vi "HFRR ADV v044.vi"() -> ()   [LabVIEW 2025] (continued)
                  selector: w401 -> [_ w412]
                  frame False {
                    w408 = TRUE ("PAUSE")
                    n303 = call "ELAPSED TIMER VI - abort test.vi"("RESET"=w408, "PAUSE"=w408) -> ()  [unwired: 7 in, 3 out]
                  }
                  frame True {
                    n304 = Not(x=w412) -> (.not. x?=w411:bool)
                    n305 = call "ELAPSED TIMER VI - abort test.vi"("TARGET"=60.0, "RESET"=w411, "PAUSE"=FALSE) -> ("ELAPSED INDICATION"=w409:bool)  [unwired: 6 in, 2 out]
                    n306 = case shown="True" w409 {
                      frame False {
                      }
                      frame True {
                        n307 = stacked-sequence {
                          frame #0 {
                            w414 = FALSE
                            n308 = local write "RUN"(w414) -> ()
                            n309 = local write "Auto Start Test"(w414) -> ()
                          }
                          frame #1 {
                            n310 = One Button Dialog(message="Test stopped due to a communication error. Reconnect the C1 and C2 cables.") -> ()  [unwired: 1 in, 1 out]
                          }
                        }
                      }
                    }
                  }
                }
              }
            }
          }
          frame Enabled {
          }
        }
        n311 = Get Date/Time In Seconds() -> (seconds since 1Jan1904=w395:timestamp)
        n312 = Format Into String(format string="%<%I:%M:%S:%p %d:%B:%Y>T", w395) -> (resulting string=→"Time Stamp":string)  [unwired: 2 in, 1 out]
        n313 = local read "Service Password enable"() -> (w387:bool)
        n314 = local read "FILE"() -> (w392:string)
        n315 = call <vilib>:"Trim Whitespace.vi"("string"=w392) -> ("trimmed string"=w391:string)  [unwired: 1 in]
        n316 = String Length(string=w391) -> (length=w390:i32)
        n317 = Greater?(x=w390, y=1) -> (0:w388:bool)
        n318 = case shown="False" w388 {
          tunnel: w387 -> [w416 _]
          frame False {
            n319 = case shown="False" w416 {
              frame True {
                w417 = "Test Start In Service Mode" ("Tip Strip")
                w418 = T19."Enabled" ("Disabled")
                n320 = property on="Auto Start Test" class="Bool (strict)"("DisabledEnum"=w418, "TipStrip"=w417) -> ()  [unwired: 2 in, 2 out]
                n321 = property on="RUN" class="Bool (strict)"("DisabledEnum"=w418, "TipStrip"=w417) -> ()  [unwired: 2 in, 2 out]
              }
              frame False {
                w419 = "Enter File Name to Start Test" ("Tip Strip")
                w420 = T19."Disabled and Grayed Out" ("Disabled")
                n322 = property on="Auto Start Test" class="Bool (strict)"("DisabledEnum"=w420, "TipStrip"=w419) -> ()  [unwired: 2 in, 2 out]
                n323 = property on="RUN" class="Bool (strict)"("DisabledEnum"=w420, "TipStrip"=w419) -> ()  [unwired: 2 in, 2 out]
              }
            }
          }
          frame True {
            w421 = "" ("Tip Strip")
            w422 = T19."Enabled" ("Disabled")
            n324 = property on="Auto Start Test" class="Bool (strict)"("DisabledEnum"=w422, "TipStrip"=w421) -> ()  [unwired: 2 in, 2 out]
            n325 = property on="RUN" class="Bool (strict)"("DisabledEnum"=w422, "TipStrip"=w421) -> ()  [unwired: 2 in, 2 out]
          }
        }
      }
      event "RUN": Value Change {
        n326 = event-data() -> ()  [unwired: 1 in, 6 out]
        n327 = local read "RUN"() -> (w424:bool)
        n328 = case shown="False" w424 {
          frame False {
            n329 = flat-sequence {
              frame #0 {
                n330 = local write "START TEMP"(FALSE ("START TEMP")) -> ()
              }
              frame #1 {
                n331 = Wait (ms)(milliseconds to wait=u32 1500) -> ()  [unwired: 1 out]
              }
              frame #2 {
                n332 = local write "Humidity 2"(TRUE ("Humidity")) -> ()
              }
              frame #3 {
                n333 = local write "Due Write"("VC;0") -> ()
              }
              frame #4 {
                n334 = Wait (ms)(milliseconds to wait=u32 1500) -> ()  [unwired: 1 out]
              }
              frame #5 {
                w434 = T19."Enabled" ("Disabled")
                (unwired) T25."Imaging" ("Main Dashboard Buttons")
                (unwired) T21."Adv Scar" ("Main Tab")
                w436 = "" ("FILE")
                n335 = local write "measured_stroke"(0.0 ("measured_stroke")) -> ()
                n336 = local write "Due Write"("VC;0") -> ()
                n337 = local write "FILE"(w436) -> ()
                n338 = local write "Batch Ref Num :"(w436) -> ()
                n339 = local write "Fuel Discription :"(w436) -> ()
                n340 = local write "Main Tab"(T4."Adv Scar" ("Main Tab")) -> ()
                n341 = local write "Remarks :"(w436) -> ()
                n342 = local write "Main Dashboard Buttons"(T1."Imaging" ("Main Dashboard Buttons")) -> ()
                n343 = local write "TEST FILE NAM,E SAVED"(FALSE ("TEST FILE NAM,E SAVED")) -> ()
                n344 = property on="Stroke ( mm )" class="WFChart (strict)"("History Data"=cluster{"y":dbl, dbl, "y":dbl}[] []) -> ()  [unwired: 2 in, 2 out]
                n345 = property on="Auto Start Test" class="Bool (strict)"("Visible"=TRUE) -> ()  [unwired: 2 in, 2 out]
                n346 = property on="FRICVALZ 2" class="Bool (strict)"("DisabledEnum"=w434) -> ()  [unwired: 2 in, 2 out]
                n347 = property on="FRICVALZ 4" class="Bool (strict)"("DisabledEnum"=w434) -> ()  [unwired: 2 in, 2 out]
                n348 = property on="FRICVALZ 3" class="Bool (strict)"("DisabledEnum"=w434) -> ()  [unwired: 2 in, 2 out]
              }
            }
          }
          frame True {
            n349 = stacked-sequence {
              frame #0 {
                n350 = local write "FRICVALZ 4"(TRUE ("FRICVALZ 4")) -> ()
                n351 = local write "Due Write"("DAC;200") -> ()
              }
              frame #1 {
              }
              frame #2 {
              }
              frame #3 {
                n352 = Wait (ms)(milliseconds to wait=u32 1000) -> ()  [unwired: 1 out]
              }
              frame #4 {
                n353 = local write "Due Write"("VC;1") -> ()
              }
              frame #5 {
                n354 = Wait (ms)(milliseconds to wait=u32 1000) -> ()  [unwired: 1 out]
              }
              frame #6 {
                n355 = local write "Due Write"("VC;1") -> ()
              }
              frame #7 {
                n356 = Wait (ms)(milliseconds to wait=u32 1500) -> ()  [unwired: 1 out]
              }
              frame #8 {
                w447 = T19."Disabled" ("Disabled")
                n357 = property on="Auto Start Test" class="Bool (strict)"("Visible"=FALSE) -> ()  [unwired: 2 in, 2 out]
                n358 = local write "START TEMP"(TRUE ("START TEMP")) -> ()
                n359 = property on="FRICVALZ 2" class="Bool (strict)"("DisabledEnum"=w447) -> ()  [unwired: 2 in, 2 out]
                n360 = property on="FRICVALZ 4" class="Bool (strict)"("DisabledEnum"=w447) -> ()  [unwired: 2 in, 2 out]
                n361 = property on="FRICVALZ 3" class="Bool (strict)"("DisabledEnum"=w447) -> ()  [unwired: 2 in, 2 out]
              }
            }
          }
        }
      }
      event "run test Calibration": Value Change {
        n362 = event-data() -> ()  [unwired: 1 in, 6 out]
        n363 = local read "run test Calibration"() -> (w449:bool)
        n364 = case shown="False" w449 {
          frame False {
            n365 = flat-sequence {
              frame #0 {
                n366 = local write "START TEMP"(FALSE ("START TEMP")) -> ()
              }
              frame #1 {
                n367 = Wait (ms)(milliseconds to wait=u32 1500) -> ()  [unwired: 1 out]
              }
              frame #2 {
              }
              frame #3 {
                n368 = local write "Due Write"("VC;0") -> ()
              }
              frame #4 {
                n369 = Wait (ms)(milliseconds to wait=u32 1500) -> ()  [unwired: 1 out]
              }
              frame #5 {
                n370 = local write "Due Write"("VC;0") -> ()
                n371 = property on="Tab Control 6" class="TabCtl (strict)"("Visible"=FALSE) -> ()  [unwired: 2 in, 2 out]
                n372 = local write "Friction Force Calibration Result Tab"(enum32{"Calibration Results", "Page 2"}."Calibration Results" ("Friction Force Calibration Result Tab")) -> ()
                n373 = property on="Friction Force Calibration Result Tab" class="TabCtl (strict)"("Visible"=TRUE) -> ()  [unwired: 2 in, 2 out]
              }
            }
          }
          frame True {
            n374 = flat-sequence {
              frame #0 {
                n375 = local write "Due Write"("VC;1") -> ()
              }
              frame #1 {
                n376 = Wait (ms)(milliseconds to wait=u32 1000) -> ()  [unwired: 1 out]
              }
              frame #2 {
                n377 = local write "Due Write"("VC;1") -> ()
              }
              frame #3 {
                n378 = Wait (ms)(milliseconds to wait=u32 2000) -> ()  [unwired: 1 out]
              }
              frame #4 {
                n379 = local write "START TEMP"(TRUE ("START TEMP")) -> ()
                n380 = property on="Tab Control 6" class="TabCtl (strict)"("Visible"=TRUE) -> ()  [unwired: 2 in, 2 out]
                n381 = local write "Friction Force Calibration Result Tab"(enum32{"Calibration Results", "Page 2"}."Calibration Results" ("Friction Force Calibration Result Tab")) -> ()
              }
            }
          }
        }
      }
      event "Auto": Value Change {
        n382 = event-data() -> ()  [unwired: 1 in, 6 out]
        n383 = stacked-sequence {
          frame #0 {
            n384 = local write "FILE"("") -> ()
          }
          frame #1 {
            n385 = Get Date/Time In Seconds() -> (seconds since 1Jan1904=w470:timestamp)
            n386 = Format Into String(format string="%<%I_%M_%S_%p_%d_%B_%Y>T", w470) -> (resulting string=w469:string)  [unwired: 2 in, 1 out]
            n387 = local write "FILE"(w469) -> ()
          }
        }
        n388 = local read "Auto"() -> (w467:bool)
        n389 = Not(x=w467) -> (.not. x?=w466:bool)
        n390 = local write "Auto"(w466) -> ()
      }
      event "Auto Start Temp": Value Change {
        n391 = event-data() -> ()  [unwired: 1 in, 6 out]
        n392 = local read "Auto Start Test"() -> (w473:bool)
        n393 = case shown="False" w473 {
          frame False {
            n394 = stacked-sequence {
              frame #0 {
                n395 = local write "START TEMP"(FALSE ("START TEMP")) -> ()
              }
              frame #1 {
                n396 = Wait (ms)(milliseconds to wait=u32 2000) -> ()  [unwired: 1 out]
              }
              frame #2 {
                n397 = local write "Due Write"("VC;0") -> ()
              }
              frame #3 {
                n398 = Wait (ms)(milliseconds to wait=u32 2000) -> ()  [unwired: 1 out]
              }
              frame #4 {
                w484 = T19."Enabled" ("Disabled")
                (unwired) T25."Imaging" ("Main Dashboard Buttons")
                w485 = "" ("FILE")
                n399 = local write "Main Tab"(T4."Adv Scar" ("Main Tab")) -> ()
                n400 = local write "measured_stroke"(0.0 ("measured_stroke")) -> ()
                n401 = local write "Main Dashboard Buttons"(T1."Imaging" ("Main Dashboard Buttons")) -> ()
                n402 = property on="RUN" class="Bool (strict)"("Visible"=TRUE) -> ()  [unwired: 2 in, 2 out]
                n403 = local write "Due Write"("VC;0") -> ()
                n404 = local write "Humidity 2"(TRUE ("Humidity")) -> ()
                n405 = local write "TEST FILE NAM,E SAVED"(FALSE ("TEST FILE NAM,E SAVED")) -> ()
                n406 = local write "Fuel Discription :"(w485) -> ()
                n407 = local write "Batch Ref Num :"(w485) -> ()
                n408 = local write "Remarks :"(w485) -> ()
                n409 = local write "FILE"(w485) -> ()
                n410 = property on="FRICVALZ 2" class="Bool (strict)"("DisabledEnum"=w484) -> ()  [unwired: 2 in, 2 out]
                n411 = property on="FRICVALZ 4" class="Bool (strict)"("DisabledEnum"=w484) -> ()  [unwired: 2 in, 2 out]
                n412 = property on="FRICVALZ 3" class="Bool (strict)"("DisabledEnum"=w484) -> ()  [unwired: 2 in, 2 out]
              }
            }
          }
          frame True {
            n413 = stacked-sequence {
              frame #0 {
                n414 = local write "Due Write"("DAC;200") -> ()
              }
              frame #1 {
                n415 = Wait (ms)(milliseconds to wait=u32 1000) -> ()  [unwired: 1 out]
              }
              frame #2 {
              }
              frame #3 {
              }
              frame #4 {
                n416 = local write "Due Write"("VC;1") -> ()
              }
              frame #5 {
                n417 = Wait (ms)(milliseconds to wait=u32 1000) -> ()  [unwired: 1 out]
              }
              frame #6 {
                n418 = local write "Due Write"("VC;1") -> ()
              }
              frame #7 {
                n419 = Wait (ms)(milliseconds to wait=u32 1500) -> ()  [unwired: 1 out]
              }
              frame #8 {
                w494 = T19."Disabled" ("Disabled")
                n420 = property on="RUN" class="Bool (strict)"("Visible"=FALSE) -> ()  [unwired: 2 in, 2 out]
                n421 = property on="FRICVALZ 2" class="Bool (strict)"("DisabledEnum"=w494) -> ()  [unwired: 2 in, 2 out]
                n422 = property on="FRICVALZ 4" class="Bool (strict)"("DisabledEnum"=w494) -> ()  [unwired: 2 in, 2 out]
                n423 = property on="FRICVALZ 3" class="Bool (strict)"("DisabledEnum"=w494) -> ()  [unwired: 2 in, 2 out]
                "START TEMP" <- TRUE
              }
            }
          }
        }
      }
      event "FILE", "USERNAME", "USER ID": Mouse Enter {
        n424 = event-data() -> ()  [unwired: 1 in, 4 out]
        n425 = dll-call lib="kernel32.dll" fn="Wow64DisableWow64FsRedirection"("OldValue"=0) -> (error out=w501:errorcluster, "OldValue"=w499:i32)  [unwired: 4 in, 1 out]
        n426 = call <vilib>:"System Exec.vi"("run minimized? (F)"=TRUE, "error in (no error)"=w501, "command line"="C:\\Program Files\\Common Files\\Microsoft Shared\\Ink\\TabTip.exe") -> ("error out"=w500:errorcluster)  [unwired: 5 in, 3 out]
        n427 = dll-call lib="kernel32.dll" fn="Wow64EnableWow64FsRedirection"(error in=w500, "OldValue"=w499) -> ()  [unwired: 4 in, 2 out]
      }
      event "EDIT": Value Change {
        n428 = event-data() -> ()  [unwired: 1 in, 6 out]
        n429 = local read "EDIT"() -> (w502:bool)
        n430 = case shown="False" w502 {
          frame False {
            n431 = control-ref of="This VI"() -> (w519:refnum<vi>)
            n432 = property class="VI"(reference=w519) -> (reference out=w510:refnum<vi>, error out=w514:errorcluster, "Panel"=w518:refnum<vi>)  [unwired: 1 in]
            n433 = property class="Pnl"(reference=w518, error in=w514) -> (reference out=w512:refnum<vi>, error out=w515:errorcluster, "Panes[]"=w517:refnum<vi>[])
            n434 = for {
              tunnel: w517 -> [w525] mode=indexing
              tunnel: T24."Always Off" ("Horizontal Scrollbar Visibility") -> [w524]
              tunnel: w515 -> [w521]
              tunnel: [w520] -> w513
              n435 = property class="Pane"(reference=w525, error in=w521, "HorizScrollbarVisibility"=w524) -> (reference out=w522:refnum<vi>, error out=w523:errorcluster)
              n436 = Close Reference(reference=w522, error in (no error)=w523) -> (error out=w520:errorcluster)
            }
            n437 = Close Reference(reference=w512, error in (no error)=w513) -> (error out=w511:errorcluster)
            n438 = Close Reference(reference=w510, error in (no error)=w511) -> (error out=w505:errorcluster)
            "error out 7" <- w505
            n439 = call <vilib>:"Clear Errors.vi"("error in (no error)"=w505) -> ("error out"=w504:errorcluster)  [unwired: 5 in, 1 out]
            n440 = local write "Service Password enable"(FALSE ("Service Password enable")) -> ()
            n441 = call <userlib>:"Fit VI window to Largest Dec.vi"("error in (no error)"=w504, "border spacing (2 px)"=1) -> ("error out"=w509:errorcluster, "dup VI Ref"=w507:refnum<vi>)  [unwired: 4 in]
            n442 = invoke on="Invoke Node" class="VI" method="FP.Run-Time Position.Maximized"(reference=w507, error in=w509) -> (error out=w508:errorcluster)  [unwired: 2 in, 3 out]
            n443 = call <vilib>:"Clear Errors.vi"("error in (no error)"=w508) -> ()  [unwired: 5 in, 2 out]
          }
          frame True {
          }
        }
      }
      event "Heater Button": Value Change {
        n444 = event-data() -> ()  [unwired: 1 in, 6 out]
        n445 = local read "Heater Button"() -> (w526:bool)
        n446 = case shown="True" w526 {
          frame True {
            n447 = stacked-sequence {
              frame #0 {
                n448 = Wait (ms)(milliseconds to wait=u32 1500) -> ()  [unwired: 1 out]
              }
              frame #1 {
                n449 = local read "Set Temp"() -> (w528:dbl)
                n450 = Number To Fractional String(number=w528, precision (6)=i16 2) -> (F-format string=w531:string)  [unwired: 2 in]
                n451 = Concatenate Strings("ST;" ("Command"), w531) -> (w530:string)
                n452 = local write "Due Write"(w530) -> ()
              }
              frame #2 {
                n453 = Wait (ms)(milliseconds to wait=u32 1500) -> ()  [unwired: 1 out]
              }
              frame #3 {
                n454 = local write "Due Write"("HE;1" ("Command")) -> ()
              }
              frame #4 {
                n455 = Wait (ms)(milliseconds to wait=u32 1500) -> ()  [unwired: 1 out]
              }
              frame #5 {
                n456 = stacked-sequence {
                  frame #0 {
                    n457 = Wait (ms)(milliseconds to wait=u32 1500) -> ()  [unwired: 1 out]
                  }
                  frame #1 {
                    n458 = local read "Set Temp"() -> (w537:dbl)
                    n459 = Number To Fractional String(number=w537, precision (6)=i16 2) -> (F-format string=w540:string)  [unwired: 2 in]
                    n460 = Concatenate Strings("ST;" ("Command"), w540) -> (w539:string)
                    n461 = local write "Due Write"(w539) -> ()
                  }
                  frame #2 {
                    n462 = Wait (ms)(milliseconds to wait=u32 1500) -> ()  [unwired: 1 out]
                  }
                  frame #3 {
                    n463 = local write "Due Write"("HE;1" ("Command")) -> ()
                  }
                  frame #4 {
                    n464 = Wait (ms)(milliseconds to wait=u32 1500) -> ()  [unwired: 1 out]
                  }
                }
              }
            }
          }
          frame False {
            n465 = stacked-sequence {
              frame #0 {
                n466 = Wait (ms)(milliseconds to wait=u32 1500) -> ()  [unwired: 1 out]
              }
              frame #1 {
                n467 = Concatenate Strings("ST;" ("Command"), "0" ("string")) -> (w547:string)
                n468 = local write "Due Write"(w547) -> ()
              }
              frame #2 {
                n469 = Wait (ms)(milliseconds to wait=u32 1500) -> ()  [unwired: 1 out]
              }
              frame #3 {
                n470 = local write "Due Write"("HE;0" ("Command")) -> ()
              }
              frame #4 {
                n471 = Wait (ms)(milliseconds to wait=u32 1500) -> ()  [unwired: 1 out]
              }
            }
          }
        }
      }
      event "Headen Service Button": Value Change {
        n472 = event-data() -> ()  [unwired: 1 in, 6 out]
        n473 = local read "Headen Service Button"() -> (w552:bool)
        n474 = case shown="True" w552 {
          frame False {
            n475 = property on="Password 3" class="Clust (strict)"("Visible"=FALSE) -> ()  [unwired: 2 in, 2 out]
            n476 = property on="Service Password Log" class="Str"("Visible"=FALSE) -> ()  [unwired: 2 in, 2 out]
          }
          frame True {
            n477 = flat-sequence {
              tunnel: [w558] -> w555
              tunnel: w555 -> [w559]
              frame #0 {
                n478 = property on="Password 3" class="Clust (strict)"("Visible"=TRUE) -> ()  [unwired: 2 in, 2 out]
                n479 = property on="Service Password Log" class="Str"("Visible"=TRUE) -> ()  [unwired: 2 in, 2 out]
              }
              frame #1 {
                n480 = call "DIALOG BOX HFRR ADV.vi"() -> ("Continue"=w558:bool)  [unwired: 8 in, 2 out]
              }
              frame #2 {
                n481 = case shown="True" w559 {
                  frame True {
                    n482 = property on="Password 3" class="Clust (strict)"("Visible"=TRUE) -> ()  [unwired: 2 in, 2 out]
                    n483 = property on="Service Password Log" class="Str"("Visible"=TRUE) -> ()  [unwired: 2 in, 2 out]
                  }
                  frame False {
                    n484 = property on="Password 3" class="Clust (strict)"("Visible"=FALSE) -> ()  [unwired: 2 in, 2 out]
                    n485 = property on="Service Password Log" class="Str"("Visible"=FALSE) -> ()  [unwired: 2 in, 2 out]
                  }
                }
              }
            }
          }
        }
      }
      event "Password 3.Service Password": Value Change {
        n486 = event-data() -> ()  [unwired: 1 in, 6 out]
        n487 = Unbundle By Name("Password 3") -> ("Service Password"=w566:string)
        n488 = call <vilib>:"Trim Whitespace.vi"("string"=w566) -> ("trimmed string"=w564:string)  [unwired: 1 in]
        n489 = Equal?(x=w564, y="Service@123") -> (x = y?=w565:bool)
        n490 = case shown="True" w565 {
          selector: w565 -> [w570 w573]
          frame False {
            w569 = FALSE
            n491 = local write "Service Password enable"(w570) -> ()
            n492 = property on="Service Password Log" class="Str"("Visible"=TRUE) -> ()  [unwired: 2 in, 2 out]
            n493 = property on="Service Left" class="Bool (strict)"("Visible"=w569) -> ()  [unwired: 2 in, 2 out]
            n494 = property on="Service Right" class="Bool (strict)"("Visible"=w569) -> ()  [unwired: 2 in, 2 out]
            n495 = property on="Service Bottom" class="Bool (strict)"("Visible"=w569) -> ()  [unwired: 2 in, 2 out]
          }
          frame True {
            w572 = TRUE
            n496 = property on="Service Password Log" class="Str"("Visible"=FALSE) -> ()  [unwired: 2 in, 2 out]
            n497 = property on="Service Left" class="Bool (strict)"("Visible"=w572) -> ()  [unwired: 2 in, 2 out]
            n498 = property on="Service Right" class="Bool (strict)"("Visible"=w572) -> ()  [unwired: 2 in, 2 out]
            n499 = property on="Service Bottom" class="Bool (strict)"("Visible"=w572) -> ()  [unwired: 2 in, 2 out]
            "Service Password enable" <- w573
          }
        }
      }
      event "Sign In": Value Change {
        w575 = FALSE ("Visible")
        n500 = event-data() -> ()  [unwired: 1 in, 6 out]
        n501 = property on="About" class="Clust (strict)"("Visible"=w575) -> ()  [unwired: 2 in, 2 out]
        n502 = property on="Password 3" class="Clust (strict)"("Visible"=w575) -> ()  [unwired: 2 in, 2 out]
        n503 = property on="Service Password Log" class="Str"("Visible"=FALSE) -> ()  [unwired: 2 in, 2 out]
      }
      event "Info": Value Change {
        n504 = event-data() -> ()  [unwired: 1 in, 6 out]
        n505 = local read "Info"() -> (w577:bool)
        n506 = case shown="False" w577 {
          frame False {
            n507 = property on="About" class="Clust (strict)"("Visible"=FALSE) -> ()  [unwired: 2 in, 2 out]
          }
          frame True {
            n508 = property on="About" class="Clust (strict)"("Visible"=TRUE) -> ()  [unwired: 2 in, 2 out]
          }
        }
      }
      event "Calibration": Value Change {
        n509 = event-data() -> ()  [unwired: 1 in, 6 out]
        n510 = local read "Calibration"() -> (w581:bool)
        n511 = case shown="False" w581 {
          frame False {
            n512 = property on="Calibration 2" class="TabCtl (strict)"("Visible"=FALSE) -> ()  [unwired: 2 in, 2 out]
            n513 = local write "Cal Password"("" ("Cal Password")) -> ()
          }
          frame True {
            n514 = property on="Calibration 2" class="TabCtl (strict)"("Visible"=TRUE) -> ()  [unwired: 2 in, 2 out]
            n515 = local write "Cal Password"("" ("Cal Password")) -> ()
          }
        }
        n516 = property on="Wrong Password" class="Str"("Visible"=FALSE) -> ()  [unwired: 2 in, 2 out]
      }
      event "Cal Password": Value Change {
        n517 = event-data() -> ()  [unwired: 1 in, 6 out]
        n518 = local read "Cal Password"() -> (w589:string)
        n519 = call <vilib>:"Trim Whitespace.vi"("string"=w589) -> ("trimmed string"=w588:string)  [unwired: 1 in]
        n520 = Equal?(x=w588, y="Cal@321") -> (x = y?=w586:bool)
        n521 = case shown="True" w586 {
          frame False {
            n522 = property on="Wrong Password" class="Str"("Visible"=TRUE) -> ()  [unwired: 2 in, 2 out]
          }
          frame True {
            n523 = property on="Wrong Password" class="Str"("Visible"=FALSE) -> ()  [unwired: 2 in, 2 out]
            n524 = local write "Main Tab"(T4."About" ("Main Tab")) -> ()
            n525 = local write "Cal Password"("" ("Cal Password")) -> ()
            n526 = local write "Main Dashboard Buttons"(T1."About" ("Main Dashboard Buttons")) -> ()
            n527 = property on="Calibration 2" class="TabCtl (strict)"("Visible"=FALSE) -> ()  [unwired: 2 in, 2 out]
            n528 = local write "Calibration"(FALSE ("Calibration")) -> ()
          }
        }
      }
      event "Calibration Selection": Value Change {
        n529 = event-data() -> ()  [unwired: 1 in, 6 out]
        n530 = local read "Calibration Selection"() -> (w598:T10)
        n531 = case shown="\"Stroke Calibration\"" w598 {
          tunnel: [T9."Stroke" ("Main Calibration Tab") T9."Friction" ("Main Calibration Tab") T9."Main" ("Main Calibration Tab") T9."Temperature" ("Main Calibration Tab")] -> w597
          frame "Stroke Calibration" {
          }
          frame "Friction Force Calibration" {
          }
          frame Default {
          }
          frame "Temperature Calibration" {
          }
        }
        n532 = local write "Main Calibration Tab"(w597) -> ()
      }
      event "Back Stroke": Value Change {
        n533 = event-data() -> ()  [unwired: 1 in, 6 out]
        n534 = local write "Main Stroke Tab"(T11."Step 1" ("Main Stroke Tab")) -> ()
        n535 = local write "Main Calibration Tab"(T9."Main" ("Main Calibration Tab")) -> ()
        n536 = local write "Back Stroke"(FALSE ("Back Stroke")) -> ()
        n537 = local write "Calibration Selection"(T10."Default" ("Calibration Selection")) -> ()
      }
      event "Step 2 Back": Value Change {
        n538 = event-data() -> ()  [unwired: 1 in, 6 out]
        n539 = local write "Main Stroke Tab"(T11."Step 1" ("Main Stroke Tab")) -> ()
        n540 = local write "Step 2 Back"(FALSE ("Back Stroke")) -> ()
        n541 = local write "Calibration Selection"(T10."Default" ("Calibration Selection")) -> ()
      }
      event "Step 3 Back": Value Change {
        n542 = event-data() -> ()  [unwired: 1 in, 6 out]
        n543 = local write "Main Stroke Tab"(T11."Step 2" ("Main Stroke Tab")) -> ()
        n544 = local write "Step 3 Back"(FALSE ("Back Stroke")) -> ()
        n545 = local write "Calibration Selection"(T10."Default" ("Calibration Selection")) -> ()
      }
      event "Step 4 Back": Value Change {
        n546 = event-data() -> ()  [unwired: 1 in, 6 out]
        n547 = local write "Main Stroke Tab"(T11."Step 3" ("Main Stroke Tab")) -> ()
        n548 = local write "Step 4 Back"(FALSE ("Back Stroke")) -> ()
        n549 = local write "Calibration Selection"(T10."Default" ("Calibration Selection")) -> ()
      }
      event "Step 5 Back": Value Change {
        n550 = event-data() -> ()  [unwired: 1 in, 6 out]
        n551 = local write "Main Stroke Tab"(T11."Step 4" ("Main Stroke Tab")) -> ()
        n552 = local write "Step 5 Back"(FALSE ("Back Stroke")) -> ()
        n553 = local write "Calibration Selection"(T10."Default" ("Calibration Selection")) -> ()
      }
      event "Step 6 Back": Value Change {
        n554 = event-data() -> ()  [unwired: 1 in, 6 out]
        n555 = local write "Main Stroke Tab"(T11."Step 5" ("Main Stroke Tab")) -> ()
        n556 = local write "Step 6 Back"(FALSE ("Back Stroke")) -> ()
        n557 = local write "Calibration Selection"(T10."Default" ("Calibration Selection")) -> ()
      }
      event "Back Stroke step 7": Value Change {
        n558 = event-data() -> ()  [unwired: 1 in, 6 out]
        n559 = local write "Main Stroke Tab"(T11."Step 5" ("Main Stroke Tab")) -> ()
        n560 = local write "Back Stroke step 7"(FALSE ("Back Stroke")) -> ()
        n561 = local write "Calibration Selection"(T10."Default" ("Calibration Selection")) -> ()
      }
      event "Back Stroke step 8": Value Change {
        n562 = event-data() -> ()  [unwired: 1 in, 6 out]
        n563 = local write "Main Stroke Tab"(T11."Step 7" ("Main Stroke Tab")) -> ()
        n564 = local write "Back Stroke step 8"(FALSE ("Back Stroke")) -> ()
        n565 = local write "Calibration Selection"(T10."Default" ("Calibration Selection")) -> ()
      }
      event "Back Stroke 8": Value Change {
        n566 = event-data() -> ()  [unwired: 1 in, 6 out]
        n567 = local write "MOVE CARRIAGE TO"(1.0 ("MOVE CARRIAGE TO")) -> ()
        n568 = local write "Main Stroke Tab"(T11."Step 1" ("Main Stroke Tab")) -> ()
        n569 = local write "Calibration Selection"(T10."Default" ("Calibration Selection")) -> ()
        n570 = local write "Back Stroke 8"(FALSE ("Back Stroke 8")) -> ()
      }
      event "Continue Stroke": Value Change {
        n571 = event-data() -> ()  [unwired: 1 in, 6 out]
        n572 = local write "Main Stroke Tab"(T11."Step 2" ("Main Stroke Tab")) -> ()
        n573 = local write "Continue Stroke"(FALSE ("Continue Stroke")) -> ()
      }
      event "Continue Stroke step 2": Value Change {
        n574 = event-data() -> ()  [unwired: 1 in, 6 out]
        n575 = local write "Main Stroke Tab"(T11."Step 3" ("Main Stroke Tab")) -> ()
        n576 = local write "Continue Stroke step 2"(FALSE ("Continue Stroke")) -> ()
      }
      event "Continue Stroke step 3": Value Change {
        n577 = event-data() -> ()  [unwired: 1 in, 6 out]
        n578 = local write "Main Stroke Tab"(T11."Step 4" ("Main Stroke Tab")) -> ()
        n579 = local write "Continue Stroke step 3"(FALSE ("Continue Stroke")) -> ()
      }
      event "Continue Stroke step 4": Value Change {
        n580 = event-data() -> ()  [unwired: 1 in, 6 out]
        n581 = local write "Main Stroke Tab"(T11."Step 5" ("Main Stroke Tab")) -> ()
        n582 = local write "Continue Stroke step 4"(FALSE ("Continue Stroke")) -> ()
      }
      event "Continue Stroke step 5": Value Change {
        n583 = event-data() -> ()  [unwired: 1 in, 6 out]
        n584 = local write "Main Stroke Tab"(T11."Step 7" ("Main Stroke Tab")) -> ()
        n585 = local write "Continue Stroke step 5"(FALSE ("Continue Stroke")) -> ()
      }
      event "Continue Stroke step 6": Value Change {
        n586 = event-data() -> ()  [unwired: 1 in, 6 out]
        n587 = local write "Main Stroke Tab"(T11."Step 7" ("Main Stroke Tab")) -> ()
        n588 = local write "Continue Stroke step 6"(FALSE ("Continue Stroke")) -> ()
      }
      event "Continue Stroke step 7": Value Change {
        w646 = FALSE ("0.2mm")
        n589 = event-data() -> ()  [unwired: 1 in, 6 out]
        n590 = local write "0.4 mm"(w646) -> ()
        n591 = local write "0.6 mm"(w646) -> ()
        n592 = local write "1.0 mm"(w646) -> ()
        n593 = local write "1.2 mm"(w646) -> ()
        n594 = local write "0.2 2"(w646) -> ()
        n595 = local write "0.4 2"(w646) -> ()
        n596 = local write "0.6 2"(w646) -> ()
        n597 = local write "0.8 2"(w646) -> ()
        n598 = local write "1.0 2"(w646) -> ()
        n599 = local write "1.2"(w646) -> ()
        n600 = local write "0.2mm"(w646) -> ()
        n601 = local write "0.8mm"(w646) -> ()
        n602 = local write "Main Stroke Tab"(T11."Step 8" ("Main Stroke Tab")) -> ()
        n603 = local write "Continue Stroke step 7"(FALSE ("Continue Stroke")) -> ()
        n604 = local write "Stroke Test Complete"(T12."Test Progress" ("Stroke Test Complete")) -> ()
        "Position Measurment Temp" <- 4.0 ("Position Measurment Temp")
        "Calibration Tare" <- TRUE ("Calibration Tare")
        "MOVE CARRIAGE TO" <- 1.0 ("MOVE CARRIAGE TO")
      }
      event "Continue Stroke step 8": Value Change {
        n605 = event-data() -> ()  [unwired: 1 in, 6 out]
        n606 = local read "LVDT STROKE  Calibration"() -> (w651:dbl)
        n607 = local read "Position Measurment Temp"() -> (w652:dbl)
        n608 = case shown="7" w652 {
          selector: w652 -> [w657 w662 w667 w672 _ w680 w683 w684]
          tunnel: w651 -> [w653 w658 w663 w668 w674 w677 _ _]
          frame 0, Default {
            w655 = TRUE ("0.2mm")
            n609 = Increment(x=w657) -> (x+1=w656:i32)
            n610 = local write "Position Measurment Temp"(w656) -> ()
            n611 = local write "0.2mm"(w655) -> ()
            n612 = local write "0.2 2"(w655) -> ()
            n613 = local write "MOVE CARRIAGE TO"(1.0 ("MOVE CARRIAGE TO")) -> ()
            "Calibration 0.2" <- w653
          }
          frame 1 {
            w660 = TRUE ("0.4 mm")
            n614 = Increment(x=w662) -> (x+1=w661:i32)
            n615 = local write "Calibration 0.4"(w658) -> ()
            n616 = local write "Position Measurment Temp"(w661) -> ()
            n617 = local write "0.4 mm"(w660) -> ()
            n618 = local write "MOVE CARRIAGE TO"(0.6 ("MOVE CARRIAGE TO")) -> ()
            n619 = local write "0.4 2"(w660) -> ()
          }
          frame 2 {
            w665 = TRUE ("0.6 mm")
            n620 = Increment(x=w667) -> (x+1=w666:i32)
            n621 = local write "Calibration 0.6"(w663) -> ()
            n622 = local write "Position Measurment Temp"(w666) -> ()
            n623 = local write "0.6 2"(w665) -> ()
            n624 = local write "0.6 mm"(w665) -> ()
            n625 = local write "MOVE CARRIAGE TO"(0.8 ("MOVE CARRIAGE TO")) -> ()
          }
          frame 3 {
            w669 = TRUE ("0.6 mm")
            n626 = Increment(x=w672) -> (x+1=w671:i32)
            n627 = local write "Position Measurment Temp"(w671) -> ()
            n628 = local write "MOVE CARRIAGE TO"(1.0 ("MOVE CARRIAGE TO")) -> ()
            n629 = local write "0.8mm"(w669) -> ()
            n630 = local write "0.8 2"(w669) -> ()
            "Calibration 0.8" <- w668
          }
          frame 4 {
            w675 = TRUE ("0.6 mm")
            n631 = local write "Position Measurment Temp"(6.0 ("Position Measurment Temp")) -> ()
            n632 = local write "MOVE CARRIAGE TO"(1.0 ("MOVE CARRIAGE TO")) -> ()
            n633 = local write "1.0 mm"(w675) -> ()
            n634 = local write "1.0 2"(w675) -> ()
            "Calibration 1.0" <- w674
          }
          frame 5 {
            w678 = TRUE ("0.6 mm")
            n635 = Increment(x=w680) -> (x+1=w679:i32)
            n636 = local write "Position Measurment Temp"(w679) -> ()
            n637 = local write "1.2 mm"(w678) -> ()
            n638 = local write "1.2"(w678) -> ()
            "Calibration 1.2" <- w677
          }
          frame 6 {
            n639 = Increment(x=w683) -> (x+1=w682:i32)
            n640 = local write "Position Measurment Temp"(w682) -> ()
            n641 = local write "Stroke Test Complete"(T12."Stroke Points Completed" ("Stroke Test Complete")) -> ()
          }
          frame 7 {
            n642 = stacked-sequence {
              tunnel: w684 -> [w685 _ _]
              frame #0 {
                n643 = Increment(x=w685) -> (x+1=w686:i32)
                n644 = local write "Main Stroke Tab"(T11."Step 9" ("Main Stroke Tab")) -> ()
                n645 = local write "Position Measurment Temp"(w686) -> ()
                n646 = Insert Into Array(array=dbl[] [], new element #1=0.2 ("new element/subarray"), new element #2=0.4 ("new element/subarray"), new element #3=0.6 ("new element/subarray"), new element #4=0.8 ("new element/subarray"), new element #5=1.0 ("new element/subarray"), new element #6=1.2 ("new element/subarray")) -> (→"1D stroke":dbl[])  [unwired: 1 in]
                n647 = local read "Calibration 0.2"() -> (w693:dbl)
                n648 = local read "Calibration 0.4"() -> (w692:dbl)
                n649 = local read "Calibration 0.6"() -> (w691:dbl)
                n650 = local read "Calibration 0.8"() -> (w690:dbl)
                n651 = local read "Calibration 1.0"() -> (w689:dbl)
                n652 = local read "Calibration 1.2"() -> (w688:dbl)
                n653 = Insert Into Array(array=dbl[] [], new element #1=w693, new element #2=w692, new element #3=w691, new element #4=w690, new element #5=w689, new element #6=w688) -> (→"Calibrated Voltage Value":dbl[])  [unwired: 1 in]
              }
              frame #1 {
                n654 = local read "calibration values"() -> (w716:dbl[])
                n655 = local read "Calibrated Voltage Value"() -> (w718:dbl[])
                n656 = Index Array(array=w716, index #1=1 ("index"), index #2=3 ("index"), index #3=5 ("index"), index #4=7 ("index"), index #5=9 ("index"), index #6=11 ("index")) -> (element #1=w709:dbl, element #2=w708:dbl, element #3=w707:dbl, element #4=w706:dbl, element #5=w705:dbl, element #6=w704:dbl)
                n657 = local read "1D stroke"() -> (w719:dbl[])
                n658 = for {
                  tunnel: [w728] -> w717 mode=indexing
                  tunnel: w719 -> [w727] mode=indexing
                  tunnel: w718 -> [w726] mode=indexing
                  tunnel: w709 -> [w725]
                  tunnel: w708 -> [w724]
                  tunnel: w707 -> [w723]
                  tunnel: w706 -> [w722]
                  tunnel: w705 -> [w721]
                  tunnel: w704 -> [w720]
                  n659 = formula code="if (stroke == 0.2)\n{\n    if ((voltage >= REF_02 - 0.2) && (voltage <= REF_02 + 0.2))\n        status = 1;\n    else\n        status = 0;\n}\nelse if (stroke == 0.4)\n{\n    if ((voltage >= REF_04 - 0.2) && (voltage <= REF_04 + 0.2))\n        status = 1;\n    else\n        status = 0;\n}\nelse if (stroke == 0.6)\n{\n    if ((voltage >= REF_06 - 0.2) && (voltage <= REF_06 + 0.2))\n        status = 1;\n    else\n        status = 0;\n}\nelse if (stroke == 0.8)\n{\n    if ((voltage >= REF_08 - 0.2) && (voltage <= REF_08 + 0.2))\n        status = 1;\n    else\n        status = 0;\n}\nelse if (stroke == 1.0)\n{\n    if ((voltage >= REF_10 - 1) && (voltage <= REF_10 + 1))\n        status = 1;\n    else\n        status = 0;\n}\nelse if (stroke == 1.2)\n{\n    if ((voltage >= REF_12 - 0.2) && (voltage <= REF_12 + 0.2))\n        status = 1;\n    else\n        status = 0;\n}\nelse\n{\n    status = 0;\n}"("stroke"=w727, "voltage"=w726, "REF_02"=w725, "REF_04"=w724, "REF_06"=w723, "REF_08"=w722, "REF_10"=w721, "REF_12"=w720) -> ("status"=w728:dbl)
                }
                "Status" <- w717
              }
              frame #2 {
                w735 = 1.0
                n660 = local read "Status"() -> (w742:dbl[])
                n661 = Index Array(array=w742) -> (element #1=w741:dbl, element #2=w740:dbl, element #3=w739:dbl, element #4=w738:dbl, element #5=w737:dbl, element #6=w736:dbl)  [unwired: 6 in]
                n662 = Equal?(x=w740, y=w735) -> (x = y?=w733:bool)
                n663 = Equal?(x=w739, y=w735) -> (x = y?=w732:bool)
                n664 = Equal?(x=w738, y=w735) -> (x = y?=w731:bool)
                n665 = Equal?(x=w737, y=w735) -> (x = y?=w730:bool)
                n666 = Equal?(x=w736, y=w735) -> (x = y?=w729:bool)
                n667 = Equal?(x=w741, y=w735) -> (x = y?=w734:bool)
                n668 = case shown="True" w734 {
                  selector: w734 -> [w753 w754]
                  frame True {
                    n669 = local write "Point 1 - 0.2 mm"(w753) -> ()
                    n670 = property on="Point 1 - 0.2 mm" class="Bool"("Caption.Visible"=w753) -> ()  [unwired: 2 in, 2 out]
                  }
                  frame False {
                    n671 = local write "Point 1 - 0.2 mm"(w754) -> ()
                    n672 = property on="Point 1 - 0.2 mm" class="Bool"("Caption.Visible"=w754) -> ()  [unwired: 2 in, 2 out]
                  }
                }
                n673 = case shown="True" w733 {
                  selector: w733 -> [w751 w752]
                  frame True {
                    n674 = local write "Point 2 - 0.4 mm"(w751) -> ()
                    n675 = property on="Point 2 - 0.4 mm" class="Bool"("Caption.Visible"=w751) -> ()  [unwired: 2 in, 2 out]
                  }
                  frame False {
                    n676 = local write "Point 2 - 0.4 mm"(w752) -> ()
                    n677 = property on="Point 2 - 0.4 mm" class="Bool"("Caption.Visible"=w752) -> ()  [unwired: 2 in, 2 out]
                  }
                }
                n678 = case shown="True" w730 {
                  selector: w730 -> [w745 w746]
                  frame True {
                    n679 = local write "Point 5 - 1.0 mm"(w745) -> ()
                    n680 = property on="Point 5 - 1.0 mm" class="Bool"("Caption.Visible"=w745) -> ()  [unwired: 2 in, 2 out]
                  }
                  frame False {
                    n681 = local write "Point 5 - 1.0 mm"(w746) -> ()
                    n682 = property on="Point 5 - 1.0 mm" class="Bool"("Caption.Visible"=w746) -> ()  [unwired: 2 in, 2 out]
                  }
                }
                n683 = case shown="True" w732 {
                  selector: w732 -> [w749 w750]
                  frame True {
                    n684 = local write "Point 3 - 0.6 mm"(w749) -> ()
                    n685 = property on="Point 3 - 0.6 mm" class="Bool"("Caption.Visible"=w749) -> ()  [unwired: 2 in, 2 out]
                  }
                  frame False {
                    n686 = local write "Point 3 - 0.6 mm"(w750) -> ()
                    n687 = property on="Point 3 - 0.6 mm" class="Bool"("Caption.Visible"=w750) -> ()  [unwired: 2 in, 2 out]
                  }
                }
                n688 = case shown="True" w731 {
                  selector: w731 -> [w747 w748]
                  frame True {
                    n689 = local write "Point 4 - 0.8 mm"(w747) -> ()
                    n690 = property on="Point 4 - 0.8 mm" class="Bool"("Caption.Visible"=w747) -> ()  [unwired: 2 in, 2 out]
                  }
                  frame False {
                    n691 = local write "Point 4 - 0.8 mm"(w748) -> ()
                    n692 = property on="Point 4 - 0.8 mm" class="Bool"("Caption.Visible"=w748) -> ()  [unwired: 2 in, 2 out]
                  }
                }
                n693 = case shown="True" w729 {
                  selector: w729 -> [w743 w744]
                  frame True {
                    n694 = local write "Point 6 - 1.2 mm"(w743) -> ()
                    n695 = property on="Point 6 - 1.2 mm" class="Bool"("Caption.Visible"=w743) -> ()  [unwired: 2 in, 2 out]
                  }
                  frame False {
                    n696 = local write "Point 6 - 1.2 mm"(w744) -> ()
                    n697 = property on="Point 6 - 1.2 mm" class="Bool"("Caption.Visible"=w744) -> ()  [unwired: 2 in, 2 out]
                  }
                }
              }
            }
          }
        }
      }
      event "Accept & Save": Value Change {
        n698 = event-data() -> ()  [unwired: 1 in, 6 out]
        n699 = flat-sequence {
          frame #0 {
            n700 = Get Date/Time In Seconds() -> (seconds since 1Jan1904=w757:timestamp)
            n701 = Format Into String(format string="%<%I:%M:%S:%p %d:%B:%Y>T", w757) -> (resulting string=w755:string)  [unwired: 2 in, 1 out]
            n702 = local write "STROKE CALIBRATION"(w755) -> ()
          }
          frame #1 {
            n703 = local write "Save Button"(TRUE ("Save Button")) -> ()
          }
          frame #2 {
            n704 = local write "MOVE CARRIAGE TO"(1.0 ("MOVE CARRIAGE TO")) -> ()
            n705 = local write "Main Calibration Tab"(T9."Main" ("Main Calibration Tab")) -> ()
            n706 = local write "Main Stroke Tab"(T11."Step 1" ("Main Stroke Tab")) -> ()
            n707 = local write "Calibration Selection"(T10."Default" ("Calibration Selection")) -> ()
            n708 = local write "Back Stroke 8"(FALSE ("Back Stroke 8")) -> ()
          }
        }
      }
      event "TEMPERATURE STEP Back 1", "TEMPERATURE STEP Back air Temp": Value Change {
        n709 = event-data() -> ()  [unwired: 1 in, 6 out]
        n710 = stacked-sequence {
          frame #0 {
            n711 = local write "Main Calibration Tab"(T9."Main" ("Main Calibration Tab")) -> ()
            n712 = local write "Tab Control 4"(T14."Main" ("Tab Control 4")) -> ()
            n713 = local write "Temperature Selection"(T15."Default" ("Temperature Selection")) -> ()
          }
          frame #1 {
            n714 = Wait (ms)(milliseconds to wait=u32 1000) -> ()  [unwired: 1 out]
            n715 = local write "Calibration Selection"(T10."Default" ("Calibration Selection")) -> ()
          }
          frame #2 {
            n716 = local write "Due Write"("CAL;END" ("Command")) -> ()
          }
          frame #3 {
            n717 = Wait (ms)(milliseconds to wait=u32 2000) -> ()  [unwired: 1 out]
          }
          frame #4 {
            n718 = local write "Due Write"("CAL;END" ("Command")) -> ()
          }
        }
      }
      event "Temperature Continue Step 1": Value Change {
        n719 = event-data() -> ()  [unwired: 1 in, 6 out]
        n720 = stacked-sequence {
          frame #0 {
            n721 = Wait (ms)(milliseconds to wait=u32 1000) -> ()  [unwired: 1 out]
          }
          frame #1 {
            n722 = local write "Due Write"("CAL;START" ("Command")) -> ()
          }
          frame #2 {
            n723 = Wait (ms)(milliseconds to wait=u32 500) -> ()  [unwired: 1 out]
          }
          frame #3 {
            n724 = local write "Due Write"("CAL;START" ("Command")) -> ()
          }
          frame #4 {
            n725 = Wait (ms)(milliseconds to wait=u32 1000) -> ()  [unwired: 1 out]
          }
          frame #5 {
          }
          frame #6 {
          }
          frame #7 {
          }
          frame #8 {
            n726 = local write "Tab Control 4"(T14."Step 2" ("Tab Control 4")) -> ()
          }
        }
      }
      event "Temperature Continue Step air Step 1": Value Change {
        n727 = event-data() -> ()  [unwired: 1 in, 6 out]
        n728 = stacked-sequence {
          frame #0 {
            n729 = Wait (ms)(milliseconds to wait=u32 1000) -> ()  [unwired: 1 out]
          }
          frame #1 {
            n730 = local write "Due Write"("CAL;START" ("Command")) -> ()
          }
          frame #2 {
            n731 = Wait (ms)(milliseconds to wait=u32 1000) -> ()  [unwired: 1 out]
          }
          frame #3 {
            n732 = local write "Due Write"("CAL;START" ("Command")) -> ()
          }
          frame #4 {
          }
          frame #5 {
          }
          frame #6 {
          }
          frame #7 {
          }
          frame #8 {
            n733 = local write "Tab Control 4"(T14."Air Step 2" ("Tab Control 4")) -> ()
          }
        }
      }
      event "Temperature Selection": Value Change {
        n734 = event-data() -> ()  [unwired: 1 in, 6 out]
        n735 = local read "Temperature Selection"() -> (w783:T15)
        n736 = case shown="\"Sample Temperature\"" w783 {
          frame "Air Temperature" {
            n737 = local write "Tab Control 4"(T14."Air Step 1" ("Tab Control 4")) -> ()
          }
          frame "Sample Temperature" {
            n738 = local write "Tab Control 4"(T14."Step 1" ("Tab Control 4")) -> ()
          }
          frame "Default", Default {
          }
        }
      }
      event "Temperature Continue Step 2": Value Change {
        n739 = event-data() -> ()  [unwired: 1 in, 6 out]
        n740 = stacked-sequence {
          frame #0 {
            n741 = stacked-sequence {
              frame #0 {
                n742 = Wait (ms)(milliseconds to wait=u32 1500) -> ()  [unwired: 1 out]
              }
              frame #1 {
                # "CAL;A1;<true_T>"
                n743 = local read "Sensor value"() -> (→"Sample 0deg temp":dbl)
                n744 = local write "Due Write"("CAL;A1;0" ("Command")) -> ()
              }
              frame #2 {
                n745 = Wait (ms)(milliseconds to wait=u32 1500) -> ()  [unwired: 1 out]
              }
              frame #3 {
                # "CAL;A1;<true_T>"
                n746 = local write "Due Write"("CAL;A1;0" ("Command")) -> ()
              }
              frame #4 {
              }
            }
          }
          frame #1 {
            n747 = local write "Tab Control 4"(T14."Step 3" ("Tab Control 4")) -> ()
          }
        }
      }
      event "Temperature Continue Air Step 2": Value Change {
        n748 = event-data() -> ()  [unwired: 1 in, 6 out]
        n749 = stacked-sequence {
          frame #0 {
            n750 = stacked-sequence {
              frame #0 {
                n751 = Wait (ms)(milliseconds to wait=u32 1000) -> ()  [unwired: 1 out]
              }
              frame #1 {
                # "CAL;A1;<true_T>"
                n752 = local write "Due Write"("CAL;A1;0" ("Command")) -> ()
              }
              frame #2 {
                n753 = Wait (ms)(milliseconds to wait=u32 1000) -> ()  [unwired: 1 out]
              }
              frame #3 {
                # "CAL;A1;<true_T>"
                n754 = local write "Due Write"("CAL;A1;0" ("Command")) -> ()
              }
              frame #4 {
                n755 = local read "Sensor value"() -> (→"Air 0deg temp":dbl)
              }
            }
          }
          frame #1 {
            n756 = local write "Tab Control 4"(T14."Air Step 3" ("Tab Control 4")) -> ()
          }
        }
      }
      event "Temperature Continue Step 3": Value Change {
        n757 = event-data() -> ()  [unwired: 1 in, 6 out]
        n758 = stacked-sequence {
          frame #0 {
            n759 = stacked-sequence {
              frame #0 {
                n760 = Wait (ms)(milliseconds to wait=u32 1500) -> ()  [unwired: 1 out]
              }
              frame #1 {
              }
              frame #2 {
              }
              frame #3 {
                # "CAL;A1;<true_T>"
                n761 = local write "Due Write"("CAL;A1;60" ("Command")) -> ()
              }
              frame #4 {
                n762 = Wait (ms)(milliseconds to wait=u32 1000) -> ()  [unwired: 1 out]
              }
              frame #5 {
                # "CAL;A1;<true_T>"
                n763 = local read "Sensor value"() -> (→"Sample 60deg temp":dbl)
                n764 = local write "Due Write"("CAL;A1;60" ("Command")) -> ()
              }
            }
          }
          frame #1 {
            w803 = 0.0
            w804 = 60.0
            n765 = local read "Sample 0deg temp"() -> (w814:dbl)
            n766 = local read "Sample 60deg temp"() -> (w813:dbl)
            n767 = Add(x=w804, y="Temperature diff") -> (x+y=w811:dbl)
            n768 = Subtract(x=w804, y="Temperature diff") -> (x-y=w810:dbl)
            n769 = Add(x=w803, y="Temperature diff") -> (x+y=w809:dbl)
            n770 = Subtract(x=w803, y="Temperature diff") -> (x-y=w808:dbl)
            n771 = In Range and Coerce(upper limit=w811, x=w813, lower limit=w810) -> (In Range?=w807:bool)  [unwired: 1 out]
            n772 = In Range and Coerce(upper limit=w809, x=w814, lower limit=w808) -> (In Range?=w806:bool)  [unwired: 1 out]
            n773 = And(x=w807, y=w806) -> (x .and. y?=w805:bool)
            n774 = case shown="True" w805 {
              frame False {
                n775 = property on="Accept & Save sample Temperature step 4" class="Bool (strict)"("DisabledEnum"=T19."Disabled" ("Disabled")) -> ()  [unwired: 2 in, 2 out]
                n776 = local write "Sample Temperature Calibration"(enum32{"True", "Fail"}."Fail" ("Sample Temperature Calibration  2")) -> ()
              }
              frame True {
                n777 = property on="Accept & Save sample Temperature step 4" class="Bool (strict)"("DisabledEnum"=T19."Enabled" ("Disabled")) -> ()  [unwired: 2 in, 2 out]
                n778 = local write "Sample Temperature Calibration"(enum32{"True", "Fail"}."True" ("Sample Temperature Calibration  2")) -> ()
              }
            }
          }
          frame #2 {
          }
          frame #3 {
          }
          frame #4 {
          }
          frame #5 {
          }
          frame #6 {
            # "CAL;END"
          }
          frame #7 {
          }
          frame #8 {
            # "CAL;END"
          }
          frame #9 {
            n779 = local write "Tab Control 4"(T14."Step 4" ("Tab Control 4")) -> ()
          }
        }
      }
      event "Accept & Save sample Temperature step 4": Value Change {
        n780 = event-data() -> ()  [unwired: 1 in, 6 out]
        n781 = stacked-sequence {
          frame #0 {
            n782 = local write "Due Write"("CAL;SAVE" ("Command")) -> ()
          }
          frame #1 {
            n783 = Wait (ms)(milliseconds to wait=u32 1000) -> ()  [unwired: 1 out]
          }
          frame #2 {
            n784 = local write "Due Write"("CAL;SAVE" ("Command")) -> ()
          }
          frame #3 {
            n785 = Wait (ms)(milliseconds to wait=u32 1000) -> ()  [unwired: 1 out]
          }
          frame #4 {
            n786 = local write "Due Write"("CAL;END" ("Command")) -> ()
          }
          frame #5 {
            n787 = Wait (ms)(milliseconds to wait=u32 1000) -> ()  [unwired: 1 out]
          }
          frame #6 {
            n788 = local write "Due Write"("CAL;END" ("Command")) -> ()
            n789 = local write "Temperature Selection"(T15."Default" ("Temperature Selection")) -> ()
            n790 = local write "Calibration Selection"(T10."Default" ("Calibration Selection")) -> ()
            n791 = local write "Tab Control 4"(T14."Main" ("Tab Control 4")) -> ()
            n792 = local write "Main Calibration Tab"(T9."Temperature" ("Main Calibration Tab")) -> ()
          }
          frame #7 {
            n793 = Get Date/Time In Seconds() -> (seconds since 1Jan1904=w833:timestamp)
            n794 = Format Into String(format string="%<%I:%M:%S:%p %d:%B:%Y>T", w833) -> (resulting string=w831:string)  [unwired: 2 in, 1 out]
            n795 = local write "TEMPERATURE CALIBRATION"(w831) -> ()
          }
          frame #8 {
            n796 = local write "Save Button"(TRUE ("Save Button")) -> ()
            n797 = local write "Tab Control 4"(T14."Main" ("Tab Control 4")) -> ()
          }
        }
      }
      event "Accept & Save Air Temperature step 4": Value Change {
        n798 = event-data() -> ()  [unwired: 1 in, 6 out]
        n799 = stacked-sequence {
          frame #0 {
            n800 = local write "Due Write"("CAL;SAVE" ("Command")) -> ()
          }
          frame #1 {
            n801 = Wait (ms)(milliseconds to wait=u32 1000) -> ()  [unwired: 1 out]
          }
          frame #2 {
            n802 = local write "Due Write"("CAL;SAVE" ("Command")) -> ()
          }
          frame #3 {
            n803 = Wait (ms)(milliseconds to wait=u32 1000) -> ()  [unwired: 1 out]
          }
          frame #4 {
            n804 = local write "Due Write"("CAL;END" ("Command")) -> ()
          }
          frame #5 {
            n805 = Wait (ms)(milliseconds to wait=u32 1000) -> ()  [unwired: 1 out]
          }
          frame #6 {
            n806 = local write "Due Write"("CAL;END" ("Command")) -> ()
            n807 = local write "Tab Control 4"(T14."Main" ("Tab Control 4")) -> ()
            n808 = local write "Main Calibration Tab"(T9."Temperature" ("Main Calibration Tab")) -> ()
            n809 = local write "Temperature Selection"(T15."Default" ("Temperature Selection")) -> ()
            n810 = local write "Calibration Selection"(T10."Default" ("Calibration Selection")) -> ()
          }
          frame #7 {
            n811 = Get Date/Time In Seconds() -> (seconds since 1Jan1904=w849:timestamp)
            n812 = Format Into String(format string="%<%I:%M:%S:%p %d:%B:%Y>T", w849) -> (resulting string=w848:string)  [unwired: 2 in, 1 out]
            n813 = local write "TEMPERATURE CALIBRATION"(w848) -> ()
          }
          frame #8 {
            n814 = local write "Tab Control 4"(T14."Main" ("Tab Control 4")) -> ()
            n815 = local write "Save Button"(TRUE ("Save Button")) -> ()
          }
        }
      }
      event "Temperature Continue Step 6": Value Change {
        n816 = event-data() -> ()  [unwired: 1 in, 6 out]
        n817 = stacked-sequence {
          frame #0 {
            n818 = stacked-sequence {
              frame #0 {
                n819 = Wait (ms)(milliseconds to wait=u32 1000) -> ()  [unwired: 1 out]
              }
              frame #1 {
              }
              frame #2 {
              }
              frame #3 {
                # "CAL;A1;<true_T>"
                n820 = local write "Due Write"("CAL;A1;60" ("Command")) -> ()
              }
              frame #4 {
                n821 = Wait (ms)(milliseconds to wait=u32 1000) -> ()  [unwired: 1 out]
              }
              frame #5 {
                # "CAL;A1;<true_T>"
                n822 = local write "Due Write"("CAL;A1;60" ("Command")) -> ()
              }
            }
          }
          frame #1 {
            n823 = local read "Sensor value"() -> (→"Air 60deg temp":dbl)
          }
          frame #2 {
          }
          frame #3 {
          }
          frame #4 {